vi "AeroQuadConfigurator.vi"() -> ()   [LabVIEW 2009] (continued)
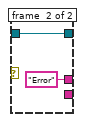
[diagram p3: hidden frame]
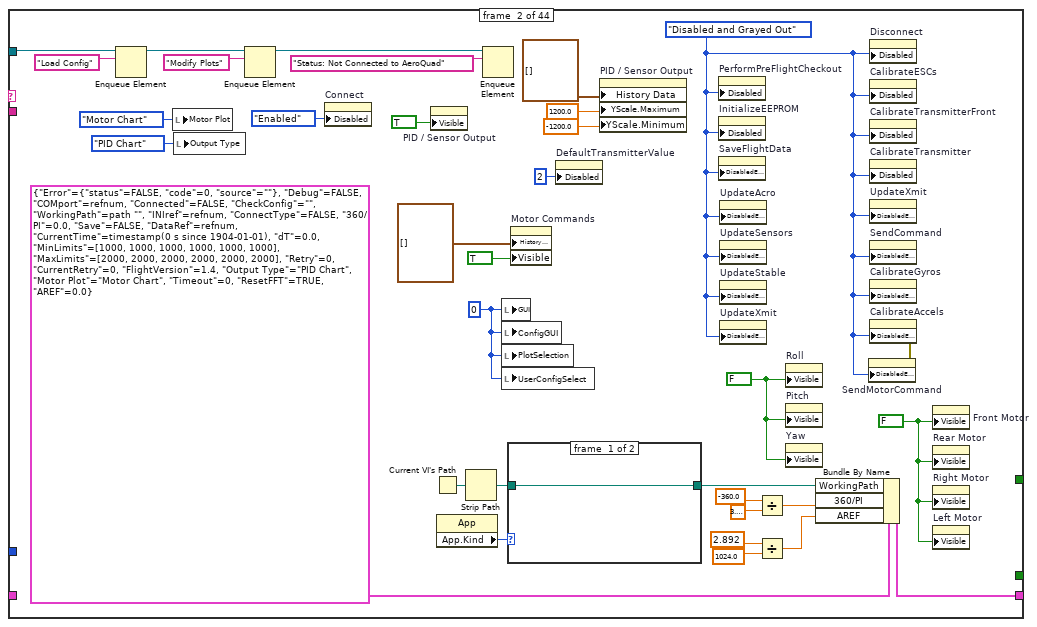
[diagram p4: hidden frame]
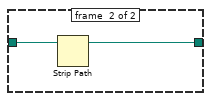
[diagram p5: hidden frame]
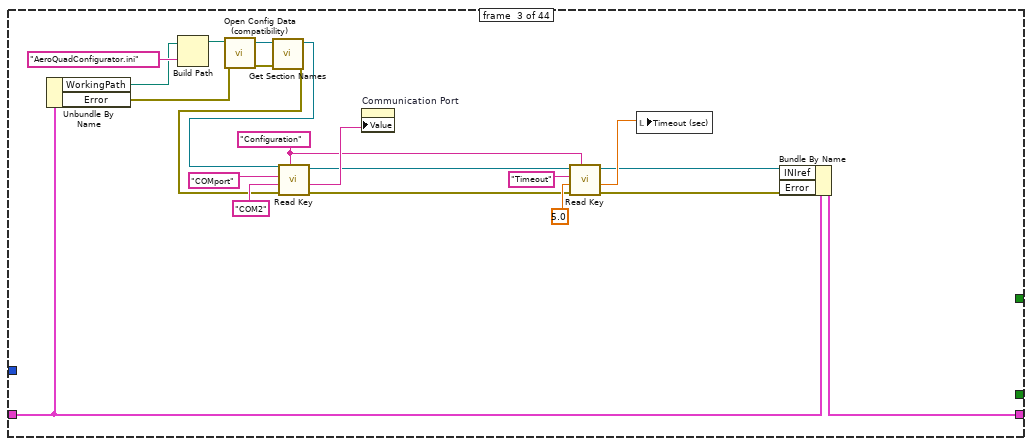
[diagram p6: hidden frame]
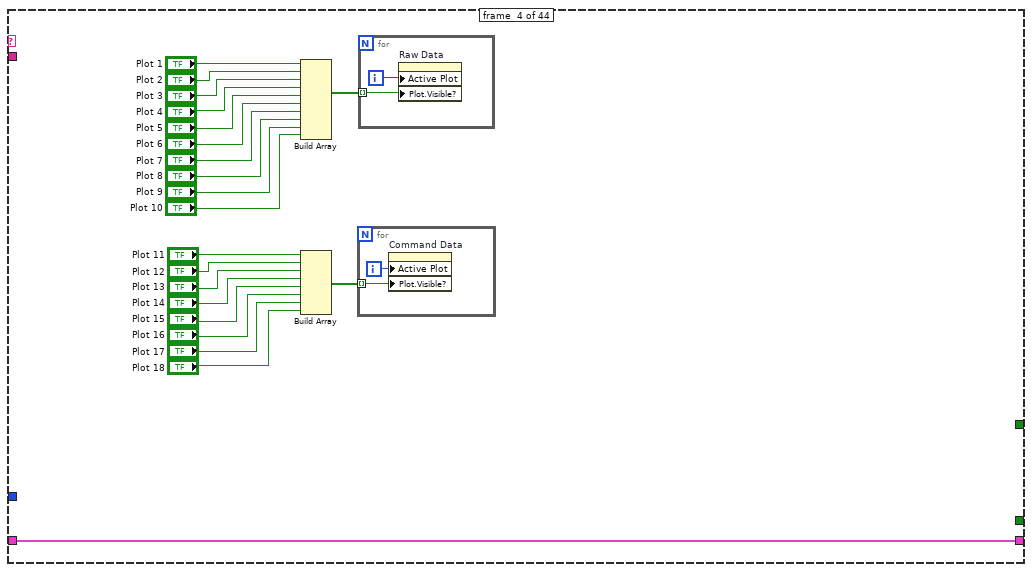
[diagram p7: hidden frame]
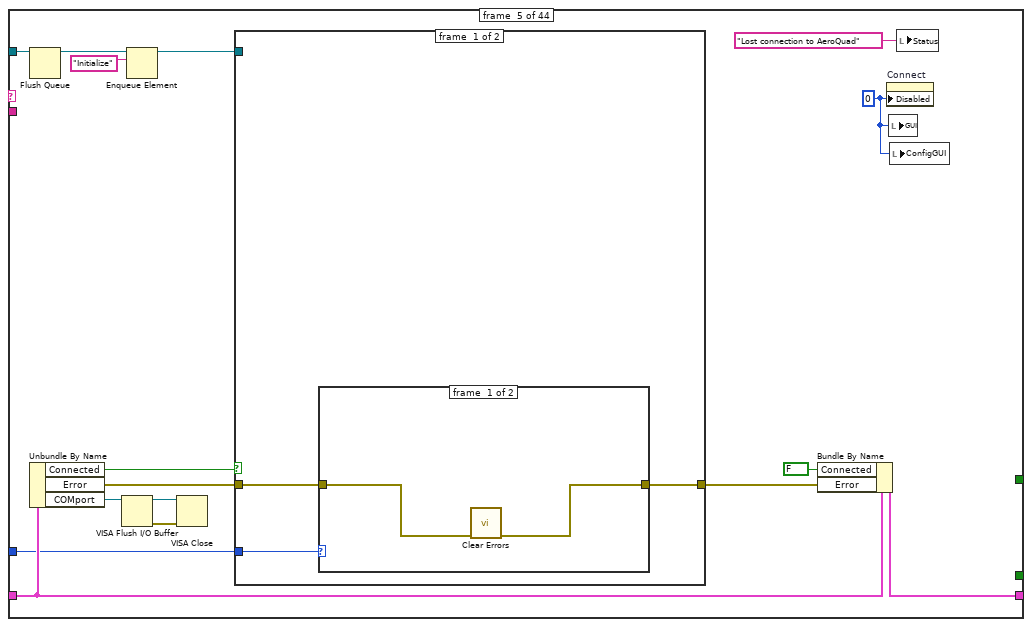
[diagram p8: hidden frame]
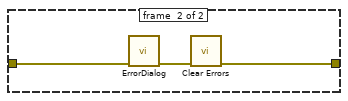
[diagram p9: hidden frame]
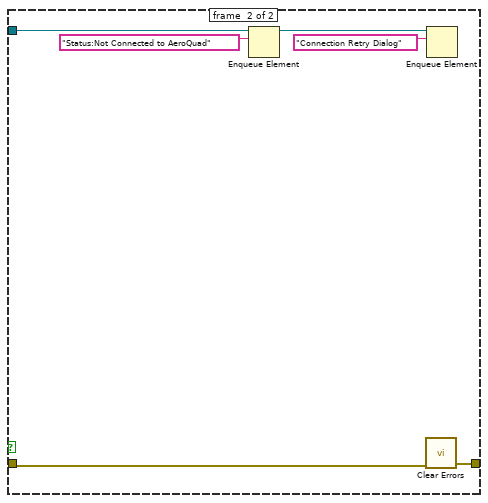
[diagram p10: hidden frame]
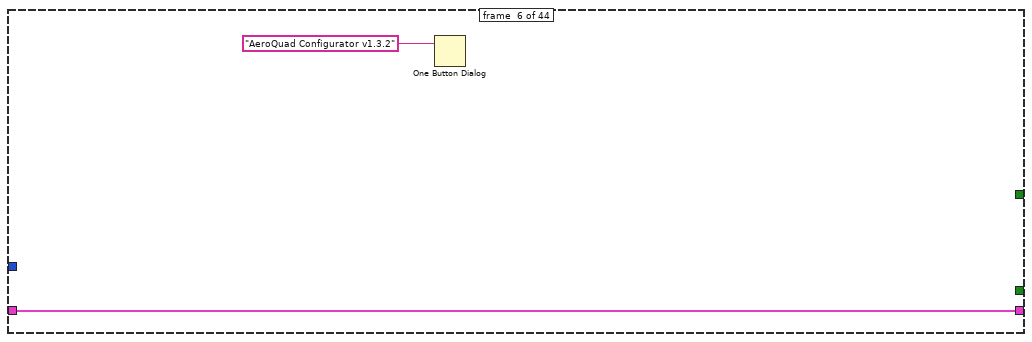
[diagram p11: hidden frame]
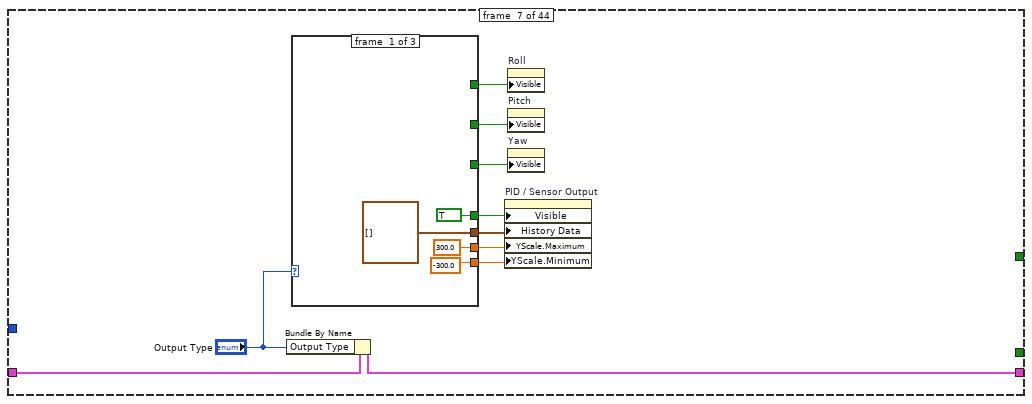
[diagram p12: hidden frame]
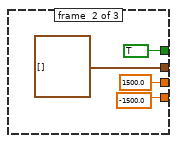
[diagram p13: hidden frame]
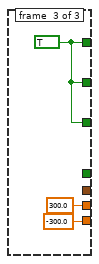
[diagram p14: hidden frame]
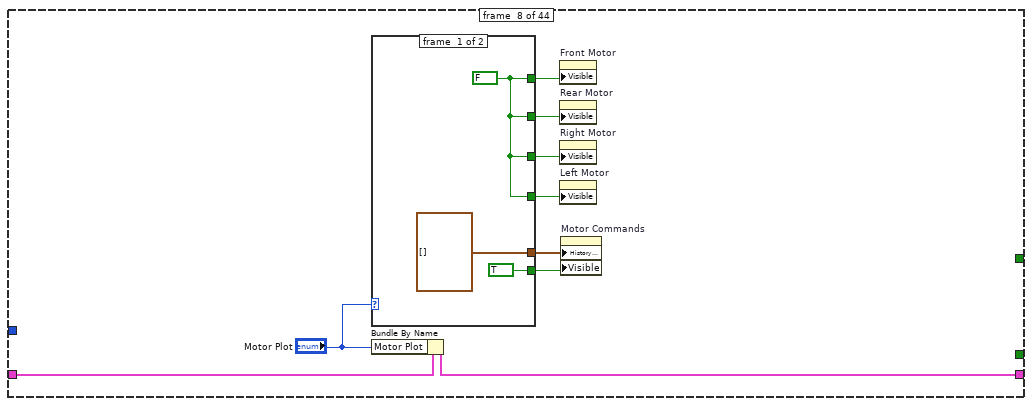
[diagram p15: hidden frame]
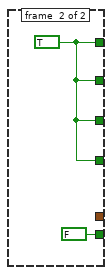
[diagram p16: hidden frame]
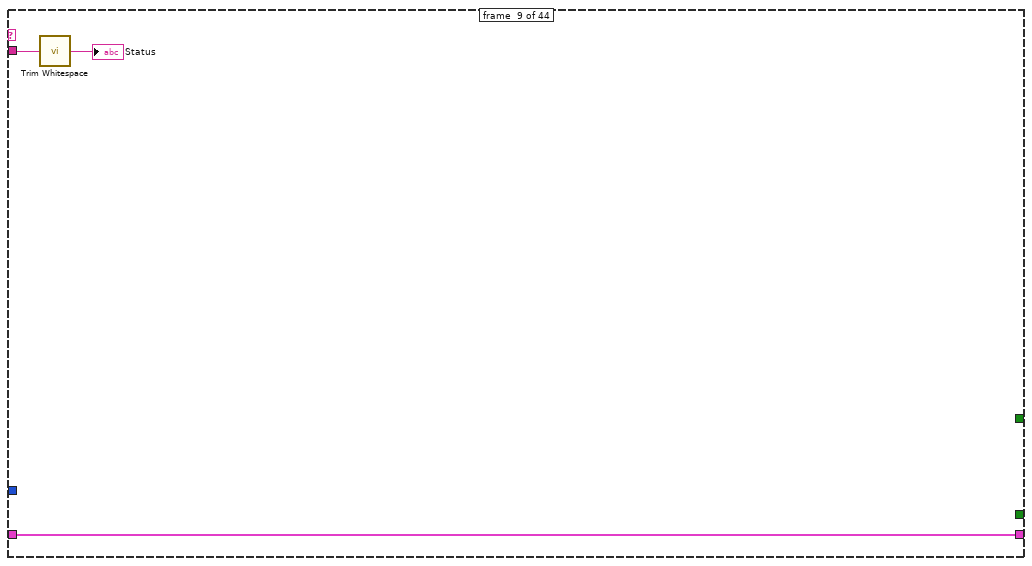
[diagram p17: hidden frame]
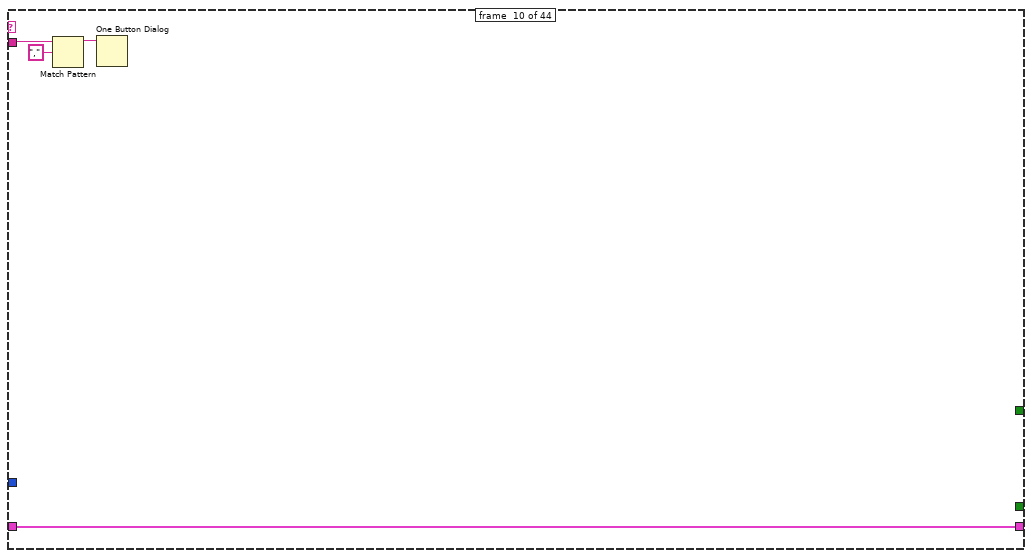
[diagram p18: hidden frame]
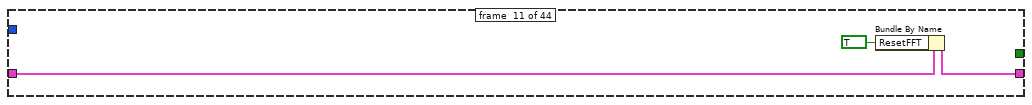
[diagram p19: hidden frame]
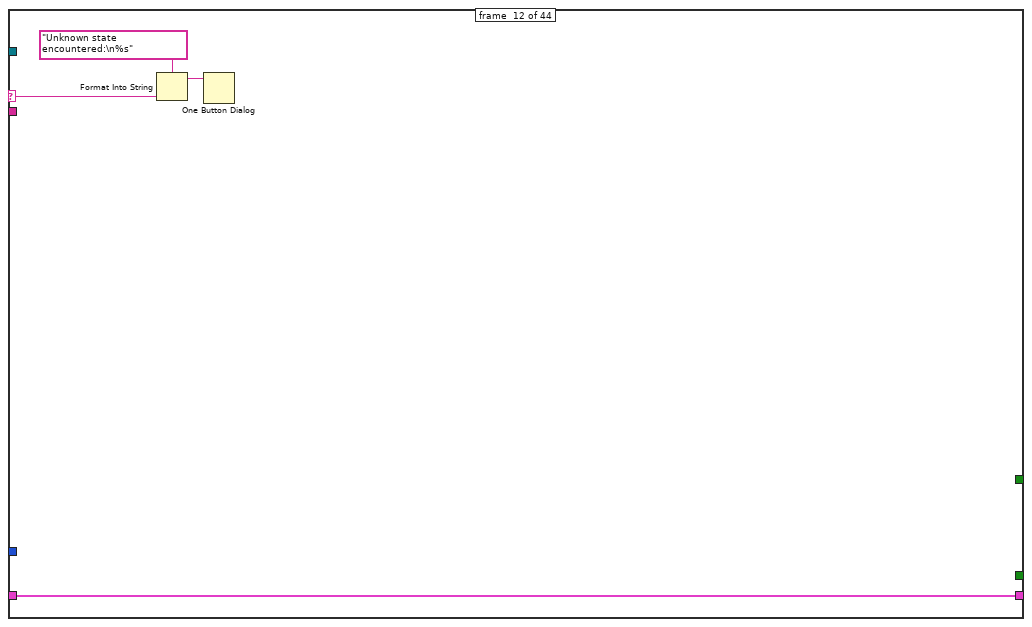
[diagram p20: hidden frame]
            n541 = local write "IntegralPitchLevel"(w1032) -> ()
            n542 = local write "DerivativePitchLevel"(w1031) -> ()
            n543 = Build Array("Level Limit", "Level Off") -> (w1040:u16[])
            n544 = call "WriteEEPROM.vi"("Write Data to EEPROM"=TRUE, "Query"="H", "Data"=w1040, "Command"="G", "error in"=w1049, "Skip"=w1051, "VISA resource name"=w1050) -> ("error out"=w1026:errorcluster, "Checked Data"=w1030:dbl[])  [unwired: 3 out]
            n545 = Index Array(array=w1030) -> (element #1=w1029:dbl, element #2=w1028:dbl)  [unwired: 2 in]
            n546 = local write "Level Limit"(w1029) -> ()
            n547 = local write "Level Off"(w1028) -> ()
            n548 = local write "Status"("Updating  Auto Level Configuration" ("Connection Status")) -> ()
          }
        }
        n549 = Bundle By Name(cluster=w1013, "Error"=w1011) -> (w1012:T11)
      }
      frame #41 {
        n550 = Unbundle By Name(w1060) -> ("COMport"=w1058:refnum<visa-resource-name>, "Connected"=w1061:bool)
        n551 = case shown="True" w1061 {
          tunnel: w1058 -> [_ w1086]
          tunnel: [_ w1070] -> w1057
          frame #0 {
          }
          frame #1 {
            w1062 = 5
            w1069 = TRUE ("Skip")
            n552 = VISA Write(VISA resource name=w1086, write buffer="X") -> (VISA resource name out=w1087:refnum<visa-resource-name>, error out=w1076:errorcluster)  [unwired: 1 in, 1 out]
            n553 = call "Time Delay12"("error in (no error)"=w1076) -> ("error out"=w1075:errorcluster)  [unwired: 1 in, 9 out]
            n554 = VISA Flush I/O Buffer(VISA resource name=w1087, error in (no error)=w1075) -> (VISA resource name out=w1077:refnum<visa-resource-name>, error out=w1074:errorcluster)  [unwired: 1 in]
            n555 = Build Array("ProportionalYaw", "IntegralYaw", "DerivativeYaw", "ProportionalHeading", "IntegralHeading", "DerivativeHeading") -> (w1073:dbl[])
            n556 = call "WriteEEPROM.vi"("Write Data to EEPROM"=w1069, "Query"="D", "Data"=w1073, "Command"="C", "error in"=w1074, "Skip"=w1069, "VISA resource name"=w1077) -> ("error out"=w1070:errorcluster, "Checked Data"=w1072:dbl[])  [unwired: 3 out]
            n557 = Index Array(array=w1072) -> (element #1=w1078:dbl, element #2=w1080:dbl, element #3=w1079:dbl, element #4=w1065:dbl, element #5=w1064:dbl, element #6=w1063:dbl)  [unwired: 6 in]
            n558 = local write "ProportionalHeading"(w1065) -> ()
            n559 = local write "IntegralHeading"(w1064) -> ()
            n560 = local write "DerivativeHeading"(w1063) -> ()
            n561 = local write "ProportionalYaw"(w1078) -> ()
            n562 = local write "IntegralYaw"(w1080) -> ()
            n563 = local write "DerivativeYaw"(w1079) -> ()
            n564 = property on="PlotSelection" class="Ring (strict)"("Value"=w1062) -> ()  [unwired: 2 in, 2 out]
            n565 = property on="GUI" class="TabCtl (strict)"("Val(Sgnl)"=w1062) -> ()  [unwired: 2 in, 2 out]
            n566 = local write "Status"("Updating Yaw Configuration" ("Connection Status")) -> ()
          }
        }
        n567 = Bundle By Name(cluster=w1060, "Error"=w1057) -> (w1059:T11)
      }
      frame #42 {
      }
      frame #43 {
        n568 = Match Pattern(string=w1101, regular expression="Enable") -> (offset past match=w1099:i32)  [unwired: 4 out]
        n569 = Unbundle By Name(w1096) -> ("DataRef"=w1094:refnum<k34>)
        n570 = Greater Or Equal To 0?(x=w1099) -> (x >= 0?=w1097:bool)
        n571 = case shown="True" w1097 {
          selector: w1097 -> [w1104 w1111]
          tunnel: [w1104 w1111] -> w1093
          tunnel: [w1102 w1127] -> w1095
          tunnel: w1094 -> [w1103 _]
          tunnel: [_ w1122] -> w1092
          tunnel: [_ w1118] -> w1091
          frame #0 {
            n572 = TDMS Close(11:w1103) -> (0:w1102:errorcluster)  [unwired: 1 in]
          }
          frame #1 {
            w1107 = path "C:/TestData" ("path (use dialog)")
            n573 = local read "Complementary Filter"() -> (w1117:dbl)
            n574 = Format Date/Time String(time format string (%c)="FlightData_%m%d%y_%H%M%S.tdms") -> (date/time string=w1113:string)  [unwired: 2 out]
            n575 = Create Folder(path (use dialog)=w1107) -> (error out=w1109:errorcluster)  [unwired: 1 in, 3 out]
            n576 = Build Path(base path=w1107, name or relative path=w1113) -> (appended path=w1112:path)
            n577 = call <vilib>:"Clear Errors.vi"("error in (no error)"=w1109) -> ("error out"=w1108:errorcluster)  [unwired: 6 out]
            n578 = Format Into String(format string="%.2f", w1117) -> (resulting string=w1115:string)  [unwired: 2 in, 1 out]
            n579 = Build Array("Test Comments", w1115, "0.100" ("element")) -> (w1119:string[])
            n580 = TDMS Open(6:FALSE ("disable buffering (T)"), 7:enum16{"1.0", "2.0"}."1.0" ("file format version (2.0)"), 8:w1108, 10:T12."create or replace" ("operation (0:open)"), 11:w1112) -> (0:w1121:errorcluster, 3:w1123:refnum<k34>)  [unwired: 1 in]
            n581 = TDMS Set Properties(5:w1119, 7:string[] ["Test Comments", "Complementary Filter Time Constant", "Delta Time In Seconds"] ("property names"), 8:w1121, 11:w1123) -> (0:w1124:errorcluster, 3:w1122:refnum<k34>)  [unwired: 4 out]
            n582 = call <vilib>:"Simple Error Handler.vi"("error in (no error)"=w1124) -> ("error out"=w1127:errorcluster)  [unwired: 1 in, 7 out]
            n583 = Get Date/Time In Seconds() -> (seconds since 1Jan1904=w1118:timestamp)
          }
        }
        n584 = Bundle By Name(cluster=w1096, "CurrentTime"=w1091, "dT"=0.0, "Save"=w1093, "DataRef"=w1092, "Error"=w1095) -> (w1098:T11)
      }
    }
  }
  n585 = while {
    tunnel: w4 -> [w1129]
    stop <- w1128 stop-if-true
    n586 = event shown="[16] \"PlotSelection\": Value Change" {
      selector: _ -> [_ _ _ _ _ _ _ _ _ _ _ _ _ _ _ _ _ _ _ _ _ _ _ _ _ _ _ _ _ _ _]
      dyn-events: _ -> [_ _ _ _ _ _ _ _ _ _ _ _ _ _ _ _ _ _ _ _ _ _ _ _ _ _ _ _ _ _ _]
      timeout: _ -> [_ _ _ _ _ _ _ _ _ _ _ _ _ _ _ _ _ _ _ _ _ _ _ _ _ _ _ _ _ _ _]
      tunnel: w1129 -> [w1135 w1143 w1156 w1158 w1191 w1193 w1195 w1196 w1202 w1209 w1231 w1245 _ w1249 w1259 _ _ _ w1284 _ w1289 w1297 w1300 w1303 w1309 w1323 _ w1329 w1337 w1345 w1348]
      tunnel: [w1130 w1141 _ _ _ _ _ _ _ _ _ _ _ _ _ _ _ _ _ _ _ _ _ _ _ _ _ _ _ _ _] -> w1128
      event #0 {
        n587 = event-data() -> ()  [unwired: 2 out]
        n588 = Two Button Dialog(message="Are you sure you want to exit?", 1:"Don't Exit" ("F button name (\"Cancel\")"), 2:"Exit" ("T button name (\"OK\")")) -> (T button?=w1131:bool)
        n589 = case shown="True" w1131 {
          tunnel: w1135 -> [_ w1138]
          tunnel: [_ TRUE] -> w1130
          frame #0 {
          }
          frame #1 {
            n590 = Flush Queue(queue=w1138) -> (queue out=w1137:refnum<queue>)  [unwired: 1 in, 2 out]
            n591 = Enqueue Element(queue=w1137, element="Exit") -> ()  [unwired: 1 in, 4 out]
          }
        }
        n592 = event-data("Discard?"=TRUE) -> ()  [unwired: 1 in, 1 out]
      }
      event #1 {
        n593 = event-data() -> ("ItemTag"=w1142:string)  [unwired: 1 out]
        n594 = case shown="\"Exit\"" w1142 {
          selector: w1142 -> [w1144 _]
          tunnel: w1143 -> [w1145 w1147]
          tunnel: [_ w1146] -> w1141
          frame #0 {
            n595 = Enqueue Element(queue=w1145, element=w1144) -> ()  [unwired: 1 in, 4 out]
          }
          frame #1 {
            n596 = Two Button Dialog(message="Are you sure you want to exit?", 1:"Exit" ("F button name (\"Cancel\")"), 2:"Continue" ("T button name (\"OK\")")) -> (T button?=w1148:bool)
            n597 = case shown="False" w1148 {
              tunnel: w1147 -> [w1154 _]
              tunnel: [TRUE _] -> w1146
              frame #0 {
                n598 = Enqueue Element(queue=w1154, element="Exit") -> ()  [unwired: 1 in, 4 out]
              }
              frame #1 {
              }
            }
          }
        }
      }
      event #2 {
        n599 = event-data() -> ()  [unwired: 2 out]
        n600 = Flush Queue(queue=w1156) -> (queue out=w1155:refnum<queue>)  [unwired: 1 in, 2 out]
        n601 = Enqueue Element(queue=w1155, element="Update Sensor Configuration") -> ()  [unwired: 1 in, 4 out]
      }
      event #3 {
        n602 = event-data() -> ()  [unwired: 2 out]
        n603 = Flush Queue(queue=w1158) -> (queue out=w1159:refnum<queue>)  [unwired: 1 in, 2 out]
        n604 = case shown="\"Flight Configuration\"" "GUI" {
          tunnel: w1159 -> [_ w1161 w1166 w1174 w1180 _ w1183 w1186]
          frame #0 {
          }
          frame #1 {
            n605 = Enqueue Element(queue=w1161, element="Configuration") -> ()  [unwired: 1 in, 4 out]
          }
          frame #2 {
            n606 = Enqueue Element(queue=w1166, element="Command:U") -> (queue out=w1164:refnum<queue>)  [unwired: 1 in, 3 out]
            n607 = Enqueue Element(queue=w1164, element="Read Transmitter Data") -> ()  [unwired: 1 in, 4 out]
            n608 = local read "Proportional Roll"() -> (w1169:dbl)
            n609 = local read "ProportionalPitch"() -> (w1167:dbl)
            n610 = Less Than 0?(x=w1169) -> (x < 0?=w1170:bool)
            n611 = Less Than 0?(x=w1167) -> (x < 0?=w1168:bool)
            n612 = property on="Roll Channel" class="Slide (strict)"("Scale.Flipped"=w1170) -> ()  [unwired: 2 in, 2 out]
            n613 = property on="Pitch Channel" class="Slide (strict)"("Scale.Flipped"=w1168) -> ()  [unwired: 2 in, 2 out]
          }
          frame #3 {
            n614 = Enqueue Element(queue=w1174, element="Command:T") -> (queue out=w1172:refnum<queue>)  [unwired: 1 in, 3 out]
            n615 = Enqueue Element(queue=w1172, element="Read Command Data") -> ()  [unwired: 1 in, 4 out]
            n616 = property on="Command Data" class="WFChart (strict)"("History Data"=T15 []) -> ()  [unwired: 2 in, 2 out]
          }
          frame #4 {
            n617 = Enqueue Element(queue=w1180, element="Command:Q") -> (queue out=w1178:refnum<queue>)  [unwired: 1 in, 3 out]
            n618 = Enqueue Element(queue=w1178, element="Read Sensor Data") -> ()  [unwired: 1 in, 4 out]
            n619 = property on="Raw Data" class="WFChart (strict)"("History Data"=T16 []) -> ()  [unwired: 2 in, 2 out]
          }
          frame #5 {
            w1181 = ""
            n620 = local write "SerialData"(w1181) -> ()
            n621 = local write "Command"(w1181) -> ()
          }
          frame #6 {
            n622 = Enqueue Element(queue=w1183, element="Command:a1;") -> (queue out=w1182:refnum<queue>)  [unwired: 1 in, 3 out]
            n623 = Enqueue Element(queue=w1182, element="Read Spectrum Analyzer") -> ()  [unwired: 1 in, 4 out]
          }
          frame #7 {
            n624 = Enqueue Element(queue=w1186, element="Command:Z") -> (queue out=w1187:refnum<queue>)  [unwired: 1 in, 3 out]
            n625 = Enqueue Element(queue=w1187, element="Read Yaw Data") -> ()  [unwired: 1 in, 4 out]
          }
        }
      }
      event #4 {
        n626 = event-data() -> ()  [unwired: 2 out]
        n627 = Enqueue Element(queue=w1191, element="Save Connect Data") -> ()  [unwired: 1 in, 4 out]
      }
      event #5 {
        n628 = event-data() -> ()  [unwired: 2 out]
        n629 = Enqueue Element(queue=w1193, element="Change Sensor Output") -> ()  [unwired: 1 in, 4 out]
      }
      event #6 {
        n630 = event-data() -> ()  [unwired: 2 out]
        n631 = Enqueue Element(queue=w1195, element="Change Motor Output") -> ()  [unwired: 1 in, 4 out]
      }
      event #7 {
        n632 = event-data() -> ()  [unwired: 2 out]
        n633 = Enqueue Element(queue=w1196, element="Modify Plots") -> ()  [unwired: 1 in, 4 out]
      }
      event #8 {
        n634 = event-data() -> ()  [unwired: 2 out]
        n635 = Two Button Dialog(message="Are you sure you want to disconnect?", 1:"Stay Connected" ("F button name (\"Cancel\")"), 2:"Disconnect" ("T button name (\"OK\")")) -> (T button?=w1198:bool)
        n636 = case shown="True" w1198 {
          tunnel: w1202 -> [_ w1203]
          frame #0 {
          }
          frame #1 {
            n637 = Flush Queue(queue=w1203) -> (queue out=w1204:refnum<queue>)  [unwired: 1 in, 2 out]
            n638 = Enqueue Element(queue=w1204, element="Status:Disconnected from AeroQuad") -> (queue out=w1205:refnum<queue>)  [unwired: 1 in, 3 out]
            n639 = Enqueue Element(queue=w1205, element="Disconnect") -> ()  [unwired: 1 in, 4 out]
          }
        }
      }
      event #9 {
        n640 = event-data() -> ("VKey"=w1210:T17, "Char"=w1208:i16)  [unwired: 1 out]
        n641 = case shown="\"Return\"" w1210 {
          tunnel: w1209 -> [_ w1212 w1213 w1224]
          tunnel: w1208 -> [_ _ _ _]
          frame #0 {
          }
          frame #1 {
            n642 = Enqueue Element(queue=w1212, element="Open COM Port") -> ()  [unwired: 1 in, 4 out]
          }
          frame #2 {
            n643 = local read "GUI"() -> (w1214:T2)
            n644 = case shown="\"Serial Monitor\"" w1214 {
              tunnel: w1213 -> [_ w1218]
              frame #0 {
              }
              frame #1 {
                n645 = local read "Command"() -> (w1215:string)
                n646 = call <vilib>:"Trim Whitespace.vi"("string"=w1215) -> ("trimmed string"=w1216:string)  [unwired: 1 in]
                n647 = Format Into String(format string="Serial Monitor Command:%s", w1216) -> (resulting string=w1219:string)  [unwired: 2 in, 1 out]
                n648 = Enqueue Element(queue=w1218, element=w1219) -> (queue out=w1217:refnum<queue>)  [unwired: 1 in, 3 out]
                n649 = flat-sequence {
                  tunnel: w1217 -> [_]
                  frame #0 {
                    n650 = local write "Command"("") -> ()
                    n651 = property on="Command" class="Str"("Key Focus"=TRUE) -> ()  [unwired: 2 in, 2 out]
                  }
                }
              }
            }
          }
          frame #3 {
            n652 = Flush Queue(queue=w1224) -> (queue out=w1223:refnum<queue>)  [unwired: 1 in, 2 out]
            n653 = Enqueue Element At Opposite End(queue=w1223, element="Disconnect") -> ()  [unwired: 1 in, 4 out]
          }
        }
      }
      event #10 {
        w1227 = u16 2 items=["Flight Configuration", "Raw Sensor Data", "Transmitter Adjustment", "Command Data", "Serial Monitor"] ("PlotSelection")
        n654 = event-data() -> ()  [unwired: 2 out]
        n655 = Flush Queue(queue=w1231) -> (queue out=w1230:refnum<queue>)  [unwired: 1 in, 2 out]
        n656 = Enqueue Element(queue=w1230, element="Initialize Transmitter") -> (queue out=w1229:refnum<queue>)  [unwired: 1 in, 3 out]
        n657 = One Button Dialog(message="Step 1:  Check that the transmitter sticks move in the same direction as on the Transmitter Adjustment screen.  If any channels move backwards, use the channel reversing function on your transmitter to make the direction match. Example: If the pitch stick is moved up, the pitch indicator in the Configurator should move up as well, not down.\n\nStep 2: For Futaba users only - Manually set the EPA for Mode (typically channel 5) and Aux (typically channel 6) to 50% at both the maximum and minimum ends.\n\nStep 3: Move both transmitter sticks to each of it's four corners (upper left, upper right, lower left, lower right). Wait a second or two at each extreme to be sure to capture the farthest position.\n\nStep 4: Flip any transmitter switches assigned to Mode or Aux to all positions. (If your transmitter is setup in Helicopter Mode, it is normal that the Aux channel moves with the Throttle channel.  If you want to customize the code to assign the Aux channel to a switch, configure your transmitter for Airplane Mode.\n\nStep 5: Feel free to move this dialog box around to view the Configurator screen. Press OK when finished.") -> (true=w1233:bool)  [unwired: 1 out]
        n658 = case shown="True" w1233 {
          tunnel: w1229 -> [w1238 _]
          frame #0 {
            n659 = Enqueue Element(queue=w1238, element="Calibrate Transmitter") -> (queue out=w1237:refnum<queue>)  [unwired: 1 in, 3 out]
            n660 = Enqueue Element(queue=w1237, element="Command:U") -> (queue out=w1235:refnum<queue>)  [unwired: 1 in, 3 out]
            n661 = Enqueue Element(queue=w1235, element="Read Transmitter Data") -> ()  [unwired: 1 in, 4 out]
          }
          frame #1 {
          }
        }
        n662 = local write "GUI"(2) -> ()
        n663 = property on="PlotSelection" class="Ring (strict)"("Value"=w1227) -> ()  [unwired: 2 in, 2 out]
      }
      event #11 {
        n664 = event-data() -> ()  [unwired: 2 out]
        n665 = Flush Queue(queue=w1245) -> (queue out=w1244:refnum<queue>)  [unwired: 1 in, 2 out]
        n666 = Enqueue Element(queue=w1244, element="Command:Y,W") -> (queue out=w1243:refnum<queue>)  [unwired: 1 in, 3 out]
        n667 = Enqueue Element(queue=w1243, element="Read Configuration") -> (queue out=w1241:refnum<queue>)  [unwired: 1 in, 3 out]
        n668 = Enqueue Element(queue=w1241, element="Status:EEPROM Initialized") -> ()  [unwired: 1 in, 4 out]
      }
      event #12 {
        n669 = event-data() -> ()  [unwired: 2 out]
        n670 = One Button Dialog(message="Under construction.  Will be implemented in future version.") -> ()  [unwired: 2 out]
      }
      event #13 {
        n671 = event-data() -> ()  [unwired: 2 out]
        n672 = Flush Queue(queue=w1249) -> (queue out=w1248:refnum<queue>)  [unwired: 1 in, 2 out]
        n673 = Enqueue Element(queue=w1248, element="Calibrate ESC's") -> ()  [unwired: 1 in, 4 out]
      }
      event #14 {
        w1252 = u16 2 items=["Flight Configuration", "Raw Sensor Data", "Transmitter Adjustment", "Command Data", "Serial Monitor"] ("PlotSelection")
        n674 = event-data() -> ()  [unwired: 2 out]
        n675 = Flush Queue(queue=w1259) -> (queue out=w1257:refnum<queue>)  [unwired: 1 in, 2 out]
        n676 = Enqueue Element(queue=w1257, element="Command:O1;0;1;0;1;0;1;0;1;0;1;0;W,U") -> (queue out=w1255:refnum<queue>)  [unwired: 1 in, 3 out]
        n677 = Enqueue Element(queue=w1255, element="Reset Limits") -> (queue out=w1254:refnum<queue>)  [unwired: 1 in, 3 out]
        n678 = Enqueue Element(queue=w1254, element="Read Transmitter Data") -> ()  [unwired: 1 in, 4 out]
        n679 = local write "GUI"(2) -> ()
        n680 = property on="PlotSelection" class="Ring (strict)"("Value"=w1252) -> ()  [unwired: 2 in, 2 out]
      }
      event #15 {
        n681 = event-data() -> ()  [unwired: 2 out]
        n682 = case shown="\"Sensors\"" "ConfigGUI" {
          frame #0 {
          }
          frame #1 {
            w1261 = 0
            n683 = property on="GUI" class="TabCtl (strict)"("Val(Sgnl)"=w1261) -> ()  [unwired: 2 in, 2 out]
            n684 = property on="PlotSelection" class="Ring (strict)"("Value"=w1261) -> ()  [unwired: 2 in, 2 out]
          }
          frame #2 {
            w1262 = 0
            n685 = property on="GUI" class="TabCtl (strict)"("Val(Sgnl)"=w1262) -> ()  [unwired: 2 in, 2 out]
            n686 = property on="PlotSelection" class="Ring (strict)"("Value"=w1262) -> ()  [unwired: 2 in, 2 out]
          }
          frame #3 {
            w1263 = 1
            n687 = property on="GUI" class="TabCtl (strict)"("Val(Sgnl)"=w1263) -> ()  [unwired: 2 in, 2 out]
            n688 = property on="PlotSelection" class="Ring (strict)"("Value"=w1263) -> ()  [unwired: 2 in, 2 out]
          }
          frame #4 {
            w1264 = 3
            n689 = property on="GUI" class="TabCtl (strict)"("Val(Sgnl)"=w1264) -> ()  [unwired: 2 in, 2 out]
            n690 = property on="PlotSelection" class="Ring (strict)"("Value"=w1264) -> ()  [unwired: 2 in, 2 out]
          }
          frame #5 {
            w1265 = 1
            n691 = property on="GUI" class="TabCtl (strict)"("Val(Sgnl)"=w1265) -> ()  [unwired: 2 in, 2 out]
            n692 = property on="PlotSelection" class="Ring (strict)"("Value"=w1265) -> ()  [unwired: 2 in, 2 out]
          }
          frame #6 {
            w1266 = 5
            n693 = property on="GUI" class="TabCtl (strict)"("Val(Sgnl)"=w1266) -> ()  [unwired: 2 in, 2 out]
            n694 = property on="PlotSelection" class="Ring (strict)"("Value"=w1266) -> ()  [unwired: 2 in, 2 out]
          }
        }
      }
      event #16 {
        n695 = event-data() -> ()  [unwired: 2 out]
        n696 = property on="GUI" class="TabCtl (strict)"() -> ("Pages"=w1268:refnum<vi>[])  [unwired: 2 in, 2 out]
        n697 = for {
          tunnel: w1268 -> [w1274] mode=indexing
          tunnel: [w1273] -> w1267 mode=indexing
          n698 = property class="Page"(reference=w1274) -> ("PageLabel"=w1273:string)  [unwired: 1 in, 2 out]
        }
        n699 = property on="PlotSelection" class="Ring (strict)"() -> ("Strings []"=w1271:string[])  [unwired: 2 in, 2 out]
        n700 = Index Array(array=w1271, index="PlotSelection") -> (element=w1270:string)
        n701 = Search 1D Array(1D array=w1267, element=w1270) -> (index of element=w1269:i32)  [unwired: 1 in]
        n702 = property on="GUI" class="TabCtl (strict)"("Val(Sgnl)"=w1269) -> ()  [unwired: 2 in, 2 out]
      }
      event #17 {
        n703 = event-data() -> ()  [unwired: 4 out]
        n704 = property on="ConfigGUI" class="TabCtl (strict)"() -> ("Pages"=w1278:refnum<vi>[])  [unwired: 2 in, 2 out]
        n705 = for {
          tunnel: w1278 -> [w1282] mode=indexing
          tunnel: [w1281] -> w1277 mode=indexing
          n706 = property class="Page"(reference=w1282) -> ("PageLabel"=w1281:string)  [unwired: 1 in, 2 out]
        }
        n707 = property on="UserConfigSelect" class="Ring (strict)"() -> ("Strings []"=w1280:string[])  [unwired: 2 in, 2 out]
        n708 = Index Array(array=w1280, index="UserConfigSelect") -> (element=w1276:string)
        n709 = Search 1D Array(1D array=w1277, element=w1276) -> (index of element=w1275:i32)  [unwired: 1 in]
        n710 = property on="ConfigGUI" class="TabCtl (strict)"("Val(Sgnl)"=w1275) -> ()  [unwired: 2 in, 2 out]
      }
      event #18 {
        n711 = event-data() -> ()  [unwired: 2 out]
        n712 = Select(t="Enable Storage" ("element"), s="SaveFlightData", f="Disable Storage" ("element")) -> (s? t:f=w1285:string)
        n713 = property on="SaveFlightData" class="Bool (strict)"("Blinking"="SaveFlightData") -> ()  [unwired: 2 in, 2 out]
        n714 = Enqueue Element(queue=w1284, element=w1285) -> ()  [unwired: 1 in, 4 out]
      }
      event #19 {
        n715 = event-data() -> ()  [unwired: 2 out]
        n716 = call <vilib>:"TDMS - File Viewer.vi"("start path"=path "C:/TestData" ("file path")) -> ()  [unwired: 2 in, 5 out]
      }
      event #20 {
        n717 = event-data() -> ()  [unwired: 2 out]
        n718 = flat-sequence {
          tunnel: w1289 -> [w1293]
          frame #0 {
            n719 = call <vilib>:"Trim Whitespace.vi"("string"="Command") -> ("trimmed string"=w1291:string)  [unwired: 1 in]
            n720 = Format Into String(format string="Serial Monitor Command:%s", w1291) -> (resulting string=w1292:string)  [unwired: 2 in, 1 out]
            n721 = Enqueue Element(queue=w1293, element=w1292) -> ()  [unwired: 1 in, 4 out]
          }
          frame #1 {
            n722 = local write "Command"("") -> ()
          }
        }
      }
      event #21 {
        n723 = event-data() -> ()  [unwired: 2 out]
        n724 = Flush Queue(queue=w1297) -> (queue out=w1296:refnum<queue>)  [unwired: 1 in, 2 out]
        n725 = Enqueue Element(queue=w1296, element="Update Configuration") -> ()  [unwired: 1 in, 4 out]
      }
      event #22 {
        n726 = event-data() -> ()  [unwired: 2 out]
        n727 = Flush Queue(queue=w1300) -> (queue out=w1299:refnum<queue>)  [unwired: 1 in, 2 out]
        n728 = Enqueue Element(queue=w1299, element="Update Auto Level Configuration") -> ()  [unwired: 1 in, 4 out]
      }
      event #23 {
        n729 = event-data() -> ()  [unwired: 2 out]
        n730 = Flush Queue(queue=w1303) -> (queue out=w1302:refnum<queue>)  [unwired: 1 in, 2 out]
        n731 = Enqueue Element(queue=w1302, element="Update Transmitter Configuration") -> ()  [unwired: 1 in, 4 out]
      }
      event #24 {
        n732 = event-data() -> ()  [unwired: 2 out]
        n733 = Flush Queue(queue=w1309) -> (queue out=w1308:refnum<queue>)  [unwired: 1 in, 2 out]
        n734 = for {
          N: 4 -> [_]
          shift-right: [w1310] -> w1305
          shift-left: "Command:5" -> [w1311]
          i -> [w1315]
          n735 = case shown="3" w1315 {
            tunnel: ["FrontMotorCommand" "RearMotorCommand" "Right MotorCommand" "LeftMotorCommand"] -> w1313
            frame #0 {
            }
            frame #1 {
            }
            frame #2 {
            }
            frame #3 {
            }
          }
          n736 = Format Into String(format string="%d;", w1313) -> (resulting string=w1312:string)  [unwired: 2 in, 1 out]
          n737 = Concatenate Strings(w1311, w1312) -> (w1310:string)
        }
        n738 = Enqueue Element(queue=w1308, element=w1305) -> ()  [unwired: 1 in, 4 out]
      }
      event #25 {
        w1320 = 1000 ("LeftMotorCommand")
        n739 = event-data() -> ()  [unwired: 2 out]
        n740 = Flush Queue(queue=w1323) -> (queue out=w1322:refnum<queue>)  [unwired: 1 in, 2 out]
        n741 = Enqueue Element(queue=w1322, element="Command:51000;1000;1000;1000;") -> ()  [unwired: 1 in, 4 out]
        n742 = local write "LeftMotorCommand"(w1320) -> ()
        n743 = local write "FrontMotorCommand"(w1320) -> ()
        n744 = local write "RearMotorCommand"(w1320) -> ()
        n745 = local write "Right MotorCommand"(w1320) -> ()
      }
      event #26 {
        n746 = event-data() -> ()  [unwired: 2 out]
        n747 = case shown="1" "MotorScale" {
          tunnel: [1200.0 ("Scale.Range:Maximum") 2000.0 ("Scale.Range:Maximum")] -> w1324
          frame #0 {
          }
          frame #1 {
          }
        }
        n748 = property on="FrontMotorCommand" class="Slide (strict)"("Scale.Maximum"=w1324) -> ()  [unwired: 2 in, 2 out]
        n749 = property on="RearMotorCommand" class="Slide (strict)"("Scale.Maximum"=w1324) -> ()  [unwired: 2 in, 2 out]
        n750 = property on="Right MotorCommand" class="Slide (strict)"("Scale.Maximum"=w1324) -> ()  [unwired: 2 in, 2 out]
        n751 = property on="LeftMotorCommand" class="Slide (strict)"("Scale.Maximum"=w1324) -> ()  [unwired: 2 in, 2 out]
      }
      event #27 {
        n752 = event-data() -> ()  [unwired: 2 out]
        n753 = Flush Queue(queue=w1329) -> (queue out=w1328:refnum<queue>)  [unwired: 1 in, 2 out]
        n754 = Enqueue Element(queue=w1328, element="Update Yaw") -> ()  [unwired: 1 in, 4 out]
      }
      event #28 {
        n755 = event-data() -> ()  [unwired: 2 out]
        n756 = Flush Queue(queue=w1337) -> (queue out=w1336:refnum<queue>)  [unwired: 1 in, 2 out]
        n757 = Enqueue Element(queue=w1336, element="Command:b") -> (queue out=w1334:refnum<queue>)  [unwired: 1 in, 3 out]
        n758 = Enqueue Element(queue=w1334, element="Status:Gyros Calibrated") -> (error out=w1332:errorcluster)  [unwired: 1 in, 3 out]
        n759 = call "Time Delay13"("error in (no error)"=w1332) -> ("error out"=w1331:errorcluster)  [unwired: 10 in]
        n760 = property on="GUI" class="TabCtl (strict)"(error in=w1331, "Val(Sgnl)"=1) -> ()  [unwired: 1 in, 2 out]
      }
      event #29 {
        n761 = event-data() -> ()  [unwired: 2 out]
        n762 = Flush Queue(queue=w1345) -> (queue out=w1344:refnum<queue>)  [unwired: 1 in, 2 out]
        n763 = Enqueue Element(queue=w1344, element="Command:c") -> (queue out=w1343:refnum<queue>)  [unwired: 1 in, 3 out]
        n764 = Enqueue Element(queue=w1343, element="Status:Accelerometers Calibrated") -> (error out=w1340:errorcluster)  [unwired: 1 in, 3 out]
        n765 = call "Time Delay17"("error in (no error)"=w1340) -> ("error out"=w1339:errorcluster)  [unwired: 10 in]
        n766 = property on="GUI" class="TabCtl (strict)"(error in=w1339, "Val(Sgnl)"=1) -> ()  [unwired: 1 in, 2 out]
      }
      event #30 {
        n767 = event-data() -> ()  [unwired: 2 out]
        n768 = Enqueue Element At Opposite End(queue=w1348, element="Reset FFT") -> ()  [unwired: 2 in, 3 out]
      }
    }
  }
  n769 = case shown="False" w1 {
    frame #0 {
      n770 = invoke class="VI" method="FP.Close"() -> ()  [unwired: 3 in, 3 out]
    }
    frame #1 {
    }
  }
